vi "HFRR ADV v041.vi"() -> ()   [LabVIEW 2025] (continued)
  # "Step 2 — Disc Holder"
  # "Remove the disc holder by loosening and removing the opposing screws. Clean any fluid present in the disc holder."
  # "Step 3 — Calibration Head"
  # "Place the calibration holder in position and securely tighten the center screw."
  # "Step 4 — Calibration Holder"
  # "Place the calibration holder in position and tighten the two securing screws"
  # "Step 5 — Tare (Spring at Free Length)"
  # "Ensure the spring is at its contact (compressed) length — the micrometer head is in contact. Click Tare Sensor to zero the friction force baseline."
  # "Step 6 — Measure Friction Force"
  # "Run the Actual Test to measure Friction Force."
  # "Step 7 — CALIBRATION RESULT"
  # "Calibration completed successfully. The measured friction force is within the acceptable tolerance range of the factory calibration value."
  # "Calibration failed. The measured friction force differs from the factory calibration value . Please perform the calibration again."
  # "Spring Constant: k = 1.000 N/mm\nSpring force |F| = k Ч d"
  # "Calibrates the sample/bath temperature sensor. \nUsed for test specimen and lubricant temperature measurement."
  # "Calibrates the ambient air temperature sensor. \nUsed for environmental chamber monitoring."
  # "Set B\n60 °C\nHigh-point calibration"
  # "Set A\n0 °C\nIce-point calibration"
  # "Set B\n60 °C\nHigh-point calibration"
  # "Set A\n0 °C\nIce-point calibration"
  # "Select Temperature Sensor"
  # "Choose which temperature sensor you are calibrating. Both use the same two-\npoint procedure: 0 °C (ice-point) and 60 °C (high-point)."
  # "Step 1 — Reference Instrument Setup"
  # "Connect a calibrated reference to the DUT port. This calibration performs two sets: one at 0 °C and one at 60 °C."
  # "Set A\n0 °C\nIce-point calibration"
  # "Set B\n60 °C\nHigh-point calibration"
  # "Allow the temperature bath to stabilise for at least 2 minutes at each set-point before recording the reading."
  # "Step 2 — Set A:  0 °C Calibration"
  # "Connect the  0 °C reference connector. Wait for the temperature to stabilise. Once stable, and click Record Point."
  # "Step 3 — Set B:  60 °C Calibration"
  # "Connect the  60 °C reference connector. Wait for the temperature to stabilise. Once stable, and click Record Point."
  # "Sample Temperature Calibration Complete"
  # "Sample Temperature Calibration PASSED\nMax deviation 0.200 °C — within ±0.5 °C tolerance. Two-point correction applied (0 °C & 60 °C)."
  # "Sample  Temperature Calibration Failed\nmeasured Sample Temperature differs from the factory calibration value"
  # "Step 1 — Reference Instrument Setup"
  # "Connect a calibrated reference to the DUT port. This calibration performs two sets: one at 0 °C and one at 60 °C."
  # "Set A\n0 °C\nIce-point calibration"
  # "Set B\n60 °C\nHigh-point calibration"
  # "Allow the temperature bath to stabilise for at least 2 minutes at each set-point before recording the reading."
  # "Step 2 — Set A:  0 °C Calibration"
  # "Connect the  0 °C reference connector. Wait for the temperature to stabilise. Once stable, and click Record Point."
  # "Step 3 — Set B:  60 °C Calibration"
  # "Connect the  60 °C reference connector. Wait for the temperature to stabilise. Once stable, and click Record Point."
  # "Air Temperature Calibration Complete"
  # "Air Temperature Calibration PASSED\nMax deviation 0.200 °C — within ±0.5 °C tolerance. Two-point correction applied (0 °C & 60 °C)."
  # "Air  Temperature Calibration Failed\nmeasured Sample Temperature differs from the factory calibration value"
  # "System Control Commands\nS;1 - Starts the full automation cycle (Runs Priming-humidify till 70RH sequence first, then switches to Maintenance).\nS;0 - Stops the system immediately and enters Standby mode (Safe State: All actuators OFF).\nM;1 - Skips the priming sequence and jumps directly to Maintenance mode (PID control).\nR;1 - Resets the logic state machine and clears all errors, returning to Standby.\nService Mode (Manual Control)\nX;1 - Enters Manual Service Mode. This disables all automatic logic, sensor safety checks, and timers.\nX;0 - Exits Manual Service Mode and returns to Standby (Safe State).\nActuator Commands (Only work after sending X;1)\nP;[0-255] - Sets the Pump PWM. Note that this is Active Low (0 = Max Flow, 255 = Pump OFF).\nF;I;[0-255] - Sets the Intake Fan speed (0 = OFF, 255 = Max Speed).\nF;O;[0-255] - Sets the Exhaust Fan speed (0 = OFF, 255 = Max Speed).\nD;1 - Turns the Dehumidifier Relay ON.\nD;0 - Turns the Dehumidifier Relay OFF."
  # "%RH"
  # "ISO : WS1.4"
  # "Start test and end test log--- done\nDisable heater ON and Humidity ON during the test --- done\ntemprature and ---done\nhumidity reach log\nauto start run true logic and log\nmanual start log once"
  # "Reference Fluid Information"
  # "Note:\nMake sure to place all images in the folder \"C:\\WinDucom\\im\" before clicking on \"Import Image.\""
  # "NOTE:\nPlace all the images in the path \"C:\\WinDucom\\im\" before clicking on Import Image"
  # "Wear Scar Measurements"
  # "Reference Fluid Information"
  # "Graph :"
types:
  T1 = enum32{"Home", "Dashboard", "Imaging", "Report", "Analysis", "About", "Test Setup", "Advance", "Calibration"}
  T2 = enum32{"HOME", "Test Setup", "Acquire", "Adv Scar", "Adv Scar Report", "Compare Files", "Calibration", "About", "Advance", "Mooha"}
  T3 = enum16{"ASTM D6079", "ISO 12156", "CEC F-096-A-06", "Custom"}
  T4 = enum32{"Dashboard 1", "Dashboard 2", "Dashboard 3"}
  T5 = enum32{"COF", "Friction", "ECR", "Temperature", "Stroke"}
  T6 = enum32{"Coefficient Of Friction", "Air Temperature", "Humidity", "Stroke", "Sample Temperature", "Electrical Contact Resistance", "Frequency", "Air Temp vs Rh"}
  T7 = enum32{"Main", "Stroke", "Friction", "Temperature"}
  T8 = enum32{"Stroke Calibration", "Friction Force Calibration", "Temperature Calibration", "Default"}
  T9 = enum32{"Step 1", "Step 2", "Step 3", "Step 4", "Step 5", "Step 6", "Step 7", "Step 8", "Step 9"}
  T10 = enum32{"Test Progress", "Stroke Points Completed"}
  T11 = enum32{"Page 1", "Page 2", "Page 3", "Page 4", "Page 5", "Page 6", "Page 7"}
  T12 = enum32{"Main", "Step 1", "Step 2", "Step 3", "Step 4", "Air Step 1", "Air Step 2", "Air Step 3", "Air Step 4"}
  T13 = enum32{"Air Temperature", "Sample Temperature", "Default"}
  T14 = enum32{"COMMUNICATION", "CALIBRATION", "Temp Variables", "Camera", "WO 2465 (1)", "WO 2465 (2)", "WO 2465 (3)"}
  T15 = typedef "Auto Start enum.ctl" = enum16{"Init", "Humidity & Temperature On", "Reach point", "Maintain Stage", "Start Stage", "close", "Exit"}
  T16 = typedef "imagedata.ctl" = cluster{"image type":i32, "image depth":i32, "image":u8[], "mask":u8[], "colors":u32[], "Rectangle":cluster{"left":i16, "top":i16, "right":i16, "bottom":i16}}
  T17 = enum32{"HOME", "Test Setup", "Acquire", "Compare Files", "Print Report", "About", "Advance", "Mooha"}
  T18 = cluster{"Read Heave and Surge":string, "Bytes at Heave Port":dbl, "Heave and Surge COM Port:":refnum<visa-resource-name>, "Com Port 2":refnum<visa-resource-name>, "Residual Due":string, "Heave COM Status 2":bool, "Heave COM Status":bool, "Port 2":bool, "Sway PPR":dbl, "Surge PPR":dbl, "Heave PPR":dbl, "Sway Pitch":dbl, "Surge Pitch":dbl, "Heave Pitch":dbl, "Sway Pulses/mm":dbl, "Surge Pulses/mm":dbl, "Heave Pulses/mm":dbl, "inner loop":dbl, "Read Heave and Surge 2":string, "String 36":string, "Write S":bool, "WriteCC1":string[], "Heave COM Loop":i32, "LastCom":string, "EXIT":bool, "Error Heave":errorcluster}
  T19 = enum8{"Enabled", "Disabled", "Disabled and Grayed Out"}
  T20 = cluster{"Read Uno":string, "Bytes at Heave Port":dbl, "UNO COM Port:":refnum<visa-resource-name>, "UNO COM Port: 2":refnum<visa-resource-name>, "Residual Due":string, "UNO COM Status 2":bool, "UNO COM Status":bool, "Port 2":bool, "Sway PPR":dbl, "Surge PPR":dbl, "Heave PPR":dbl, "Sway Pitch":dbl, "Surge Pitch":dbl, "Heave Pitch":dbl, "Sway Pulses/mm":dbl, "Surge Pulses/mm":dbl, "Heave Pulses/mm":dbl, "inner loop":dbl, "Read Heave and Surge 2":string, "String 36":string, "Write S":bool, "WriteCC1":string[], "Heave COM Loop":i32, "LastCom":string, "EXIT":bool, "Error Heave":errorcluster}
  T21 = enum32{"HOME", "Test Setup", "Acquire", "Adv Scar", "Adv Scar Report", "Compare Files", "About", "Advance", "Mooha"}
  T22 = typedef "POST ANALYSIS ENUM.ctl" = enum16{"OPEN EXE", "INIT", "OPEN FILE", "FIT", "DRAW REC", "DRAW LINE", "PAN", "ZOOM IN", "ZOOM OUT", "SET ZOOM", "CLEAR ROI", "GET MEASUREMENTS", "RESIZE MODE", "STREAM START", "STREAM STOP", "SHOW UI", "MINIMIZE UI", "HIDE UI", "CKISE APP", "CLOSE CONNECTION", "SAVE IMAGE", "SET ROI COLOR", "READ", "TCP CHECK", "CLOSE"}
  T23 = typedef "CAMERA LIVE FEED ENUM.ctl" = enum16{"OPEN EXE", "INIT", "READ", "CAMERA CONNECT", "CAMERA START", "CAMERA STOP", "CAMERA GRAY", "CAMERA RGB", "CAMERA MINIMIZE", "CAMERA CLOSE", "CAMERA MODE LIST", "CAMERA MODE SET", "CAMERA RESTORE", "CAMERA SAVE", "CLOSE"}
  T24 = enum16{"Always On", "Always Off", "Off While Running"}
  T25 = enum32{"Page 1", "Page 2", "Page 3", "Page 4", "Page 5", "Page 6"}
  T26 = enum32{"Home", "Dashboard", "Imaging", "Report", "Analysis", "About", "Test Setup", "Advance"}
  T27 = cluster{"File Name":string, "Test Method":string, "Operator":string, "Fuel Description":string, "Date and time":string}
  T28 = enum32{"Home", "Dashboard", "Imaging", "Report", "Analysis", "About", "Test Setup"}
  T29 = enum32{"HOME", "Test Setup", "Acquire", "Compare Files", "About", "Advance", "Mooha"}
  T30 = typedef "NI_ReportGenerationCore.lvlib/HTML Report Image Alignment.ctl" = enum16{"(default)", "LEFT", "RIGHT", "TOP", "TEXTTOP", "MIDDLE", "ABSMIDDLE", "BASELINE", "BOTTOM", "ABSBOTTOM"}
  T31 = cluster{"y":dbl, "LVDT STROKE DISPLAY":dbl, "y":dbl}
  T32 = enum16{"INIT", "READ", "MANUAL WRITE", "WRITE", "CLOSE", "ERROR INIT"}
diagram:
  w5 = 0.0 ("ch0_filt")
  w7 = -9999999.0 ("max_ch0")
  w8 = 9999999.0 ("min_ch0")
  w19 = FALSE ("Visible")
  w20 = T19."Enabled" ("Disabled")
  w23 = FALSE ("Visible")
  w22 = FALSE ("Humidity Off Command")
  w38 = "" ("USER ID")
  (unwired) T21."HOME" ("Main Tab")
  # "Temperature Continue Air Step 2"
  # "[CH1]    - FF\n[CH2]   - TEMPERATURE\n[CH3]    - Humidity\n[CH4]    - AIR TEMP\n[CH5]\\- Visa Uno\n[CH6] \\- Visa Due\n[CH7]  \\- file path\n[CH8]   - Displacement Gain\n[CHA]   - Stroke Gain\n[CHB]   - Stroke PID Gain\n[CHC]   -Language Selection\n[CHD]   -Power +\n[CHE]   -Power_\n[CHF]   -Heater\n[CHG]   -Humidity Wet\n[CHH]   -Humidity Dry\n[CHI]   -Integral Time \n[CHIJ   -Air intercept\n[CHI]   -Temp Intercept"
  n1 = local write "Cal Password"("" ("Cal Password")) -> ()
  n2 = property on="Auto Start Test" class="Bool (strict)"("Visible"=TRUE) -> ()  [unwired: 2 in, 2 out]
  n3 = property on="FRICVALZ 2" class="Bool (strict)"("DisabledEnum"=w20) -> ()  [unwired: 2 in, 2 out]
  n4 = property on="FRICVALZ 4" class="Bool (strict)"("DisabledEnum"=w20) -> ()  [unwired: 2 in, 2 out]
  n5 = property on="FRICVALZ 3" class="Bool (strict)"("DisabledEnum"=w20) -> ()  [unwired: 2 in, 2 out]
  n6 = property on="About" class="Clust (strict)"("Visible"=FALSE) -> ()  [unwired: 2 in, 2 out]
  n7 = property on="Wrong Password" class="Str"("Visible"=w19) -> ()  [unwired: 2 in, 2 out]
  n8 = property on="Calibration 2" class="TabCtl (strict)"("Visible"=w19) -> ()  [unwired: 2 in, 2 out]
  n9 = local write "Temperature Selection"(T13."Default" ("Temperature Selection")) -> ()
  n10 = flat-sequence {
    tunnel: [w66] -> w4
    tunnel: [w111] -> w30
    tunnel: w4 -> [w106]
    tunnel: [w112] -> w32
    tunnel: w30 -> [w112]
    tunnel: w32 -> [w172]
    tunnel: [w172] -> w31
    tunnel: w31 -> [w203]
    tunnel: [w203] -> w41
    tunnel: w41 -> [w210]
    tunnel: [w216] -> w29
    tunnel: [w204] -> w28
    tunnel: [w258] -> w3
    tunnel: [w257] -> _
    tunnel: w29 -> [w257]
    tunnel: w28 -> [w258]
    frame #0 {
      n11 = call "CLOSE CONNECTION.vi"("error in (no error)"="error in (no error) 2") -> ("error out"=w71:errorcluster)  [unwired: 10 in]
      n12 = call <vilib>:"Clear Errors.vi"("error in (no error)"=w71) -> ("error out"=w70:errorcluster)  [unwired: 5 in, 1 out]
      n13 = disable-structure shown="Enabled" {
        disable-tunnel: w70 -> [w98 _]
        disable-tunnel: [w97 _] -> w69
        frame Enabled {
          n14 = call <userlib>:"Fit VI window to Largest Dec.vi"("error in (no error)"=w98, "border spacing (2 px)"=1) -> ("error out"=w101:errorcluster, "dup VI Ref"=w105:refnum<vi>)  [unwired: 4 in]
          n15 = invoke on="Invoke Node" class="VI" method="FP.Run-Time Position.Maximized"(reference=w105, error in=w101) -> (error out=w102:errorcluster)  [unwired: 2 in, 3 out]
          n16 = call <vilib>:"Clear Errors.vi"("error in (no error)"=w102) -> ("error out"=w104:errorcluster)  [unwired: 5 in, 1 out]
          n17 = control-ref of="This VI"() -> (w96:refnum<vi>)
          n18 = invoke on="Invoke Node" class="VI" method="Default Vals.Reinit All"(reference=w96, error in=w104) -> (reference out=w100:refnum<vi>, error out=w99:errorcluster)  [unwired: 1 in, 1 out]
          n19 = Close Reference(reference=w100, error in (no error)=w99) -> (error out=w97:errorcluster)
        }
        frame Disabled {
        }
      }
      n20 = call "Stall Data Flow.vim"("value in"=w69, "milliseconds to wait"=u32 2000) -> ("value out"=w68:errorcluster)  [unwired: 1 out]
      n21 = call "Read Config.vi"("error in (no error)"=w68) -> ("error out"=w66:errorcluster, "STROKE PARAMETERS"=w77:dbl[], "ADC PARAMETERS"=w78:dbl[], "PID  PARAMETERS"=w79:dbl[], "CALIBRATION PARAMETERS"=w64:string[], "Stroke Calibration"=w76:string)  [unwired: 5 in]
      n22 = Index Array(array=w77) -> (element #1=w94:dbl, element #2=w95:dbl)  [unwired: 2 in]
      n23 = Index Array(array=w64) -> (element #1=w63:string, element #2=w62:string, element #3=w61:string, element #4=w60:string, element #5=w59:string)  [unwired: 5 in]
      n24 = Index Array(array=w78) -> (element #1=w90:dbl, element #2=w91:dbl, element #3=w92:dbl, element #4=w93:dbl)  [unwired: 4 in]
      n25 = Index Array(array=w79) -> (element #1=w81:dbl, element #2=w82:dbl, element #3=w83:dbl, element #4=w84:dbl, element #5=w85:dbl, element #6=w86:dbl, element #7=w87:dbl, element #8=w88:dbl, element #9=w89:dbl)  [unwired: 9 in]
      n26 = local write "milliseconds to wait"(w81) -> ()
      n27 = local write "dt"(w82) -> ()
      n28 = local write "kp"(w83) -> ()
      n29 = local write "ki"(w84) -> ()
      n30 = local write "kd"(w85) -> ()
      n31 = local write "max_step_change"(w86) -> ()
      n32 = local write "max_amplitude"(w87) -> ()
      n33 = local write "min_amplitude"(w88) -> ()
      n34 = local write "startup_cmd"(w89) -> ()
      n35 = local write "VREF"(w90) -> ()
      n36 = local write "ADC_Resolution"(w91) -> ()
      n37 = local write "PIEZO_CAL_FACTOR"(w92) -> ()
      n38 = local write "NORMAL_FORCE"(w93) -> ()
      n39 = local write "STROKE FILTER"(w94) -> ()
      n40 = local write "Add up Stroke"(w95) -> ()
      n41 = local write "Machine Serial Number"(w59) -> ()
      n42 = local write "STROKE CALIBRATION"(w63) -> ()
      n43 = local write "FRICTION CALIBRATION"(w62) -> ()
      n44 = local write "TEMPERATURE CALIBRATION"(w61) -> ()
      n45 = Fract/Exp String To Number(string=w60) -> (number=w65:dbl)  [unwired: 3 in, 1 out]
      n46 = Spreadsheet String To Array(delimiter (Tab)=";", format string="", spreadsheet string=w76, array type (2D Dbl)=dbl[] []) -> (array=w80:dbl[])
      n47 = local write "Temperature diff"(w65) -> ()
      n48 = local write "calibration values"(w80) -> ()
    }
    frame #1 {
      n49 = property on="Auto Scar Check" class="Clust (strict)"("Visible"=TRUE) -> ()  [unwired: 2 in, 2 out]
      n50 = property on="Sign In" class="Bool (strict)"("DisabledEnum"=T19."Disabled" ("Disabled")) -> ()  [unwired: 2 in, 2 out]
      n51 = local write "sign in temp"(FALSE ("sign in temp")) -> ()
      n52 = call "dialog box.vi"("Status"="Before starting the test, verify that the microscope cable is connected.", "error in"=w106) -> ("error out"=w111:errorcluster)  [unwired: 8 in]
    }
    frame #2 {
      (unwired) TRUE ("Re-Initialise")
      # "kkkkk"
      # "C:\\Windows\\wndcm_pw_stdED hfrr.txt"
      # "C:\\LAB-IQ NXT"
      # "C:\\LAB-IQ NXT\\wndcm_pw_stdED hfrr.txt"
      # "password file"
      n53 = Current VI's Path() -> (path=w128:path)
      n54 = Strip Path(path=w128) -> (stripped path=w121:path)  [unwired: 1 out]
      n55 = local write "main tab sub"(enum32{"Page 1", "Page 2"}."Page 1" ("main tab sub")) -> ()
      n56 = local write "Main Tab Display"(T4."Dashboard 1" ("Main Tab Display")) -> ()
      n57 = local write "Main Tab"(T2."HOME" ("Main Tab")) -> ()
      n58 = Path To String(path=w121) -> (string=w123:string)
      n59 = Search/Split String(string=w123, search string/char (-)=".exe") -> (match + rest of string=w125:string)  [unwired: 1 in, 2 out]
      n60 = Match True/False String(2:".vi" ("false string"), 3:".exe" ("true string"), 4:w125) -> (0:w122:bool)  [unwired: 1 out]
      n61 = List Folder(path=path "C:/LAB-IQ" ("directory path"), pattern="*.txt") -> (filenames=w134:string[])  [unwired: 2 in, 3 out]
      n62 = case shown="True" w122 {
        tunnel: w121 -> [w143 w145]
        tunnel: [w143 w144] -> w119
        frame False {
        }
        frame True {
          n63 = Strip Path(path=w145) -> (stripped path=w144:path)  [unwired: 1 out]
        }
      }
      n64 = Search 1D Array(1D array=w134, element="wndcm_pw_stdED hfrr.txt") -> (index of element=w137:i32)  [unwired: 1 in]
      n65 = Equal?(x=w137, y=-1) -> (x = y?=w132:bool)
      n66 = Path To String(path=w119) -> (string=→"Gain path":string)
      n67 = case shown="True" w132 {
        frame False {
        }
        frame True {
          n68 = String To Byte Array(string="123\n") -> (unsigned byte array=w150:u8[])
          n69 = Array Size(array=w150) -> (size(s)=w149:i32)
          n70 = for {
            N: w149 -> [_]
            tunnel: w150 -> [w163]
            tunnel: [w160] -> w152 mode=indexing
            tunnel: w149 -> [w155]
            i -> [w153]
            n71 = Decrement(x=w155) -> (x-1=w156:i32)
            n72 = Index Array(array=w163, index=w153) -> (element=w162:u8)
            n73 = Equal?(x=w153, y=w156) -> (x = y?=w157:bool)
            n74 = Number To Decimal String(number=w162) -> (decimal integer string=w161:string)  [unwired: 1 in]
            n75 = Select(t="", s=w157, f="\r") -> (s? t:f=w154:string)
            n76 = Concatenate Strings(w161, w154) -> (w160:string)
          }
          n77 = local read "file path"() -> (w146:path)
          n78 = Concatenate Strings(w152) -> (w148:string)
          n79 = call <vilib>:"Write Characters To File.vi"("append to file? (new file:F)"=FALSE, "character string"=w148, "file path (dialog if empty)"=w146) -> ()  [unwired: 2 in, 1 out]
        }
      }
      n80 = local write "conststatus"(0.0 ("rpm value : 2")) -> ()
      n81 = local write "EVENT LOG"("") -> ()
      n82 = local write "COUNT"(0 ("COUNT")) -> ()
      n83 = local write "clk"(0.0 ("clk")) -> ()
      n84 = local write "Flag"(0.0 ("Flag")) -> ()
      n85 = local write "Lan flag"(0.0 ("Lan flag")) -> ()
      n86 = local write "Com flag"(u32 0 ("Com flag")) -> ()
      n87 = local write "refresh flag"(FALSE ("refresh flag")) -> ()
      "file path" <- path "C:/LAB-IQ/wndcm_pw_stdED hfrr.txt" ("file path")
      "FF buffer" <- dbl[] [] ("FF buffer")
    }
    frame #3 {
      # "C:\\WinDucom\\calibrate WO 2391.dcf"
      n88 = String To Path(string="C:\\LAB-IQ\\Image Calibrate v01.dcf") -> (path=w167:path)
      n89 = String To Path(string="C:\\LAB-IQ\\calibrate WO 2465.dcf") -> (path=w171:path)
      n90 = Open/Create/Replace File "Open File"(file path (use dialog)=w171) -> (refnum out=w170:refnum<file>)  [unwired: 5 in, 2 out]
      n91 = Open/Create/Replace File ("Open File")(file path (use dialog)=w167) -> (refnum out=w166:refnum<file>)  [unwired: 5 in, 2 out]
      n92 = for {
        N: 4 -> [_]
        tunnel: w166 -> [w178]
        i -> [w174]
        n93 = Read from Text File ("Read File")(file (use dialog)=w178) -> (text=w179:string)  [unwired: 3 in, 3 out]
        n94 = String Subset(string=w179, offset (0)=6, length (rest)=10 ("length (rest)")) -> (substring=w175:string)
        n95 = Fract/Exp String To Number(string=w175) -> (number=w173:dbl)  [unwired: 3 in, 1 out]
        n96 = case shown="3" w174 {
          tunnel: w173 -> [w180 w181 _ w182 _]
          frame 0 {
            n97 = local write "5x Gain"(w180) -> ()
          }
          frame 1 {
            n98 = local write "10x Gain"(w181) -> ()
          }
          frame 2 {
          }
          frame 3 {
            n99 = local write "100x gain"(w182) -> ()
          }
          frame 4, Default {
          }
        }
      }
      n100 = for {
        N: 24 -> [_]
        tunnel: w170 -> [w191]
        i -> [w185]
        (unwired) TRUE ("line mode (F)")
        n101 = Read from Text File "Read File"(file (use dialog)=w191) -> (text=w190:string)  [unwired: 3 in, 3 out]
        n102 = Match Pattern(string=w190, regular expression="]") -> (after substring=w188:string)  [unwired: 1 in, 3 out]
        n103 = String Subset(string=w190, offset (0)=5, length (rest)=10 ("length (rest)")) -> (substring=w183:string)
        n104 = Fract/Exp String To Number(string=w183) -> (number=w184:dbl)  [unwired: 3 in, 1 out]
        n105 = Match Pattern(string=w188, regular expression="-") -> (before substring=w186:string)  [unwired: 1 in, 3 out]
        n106 = case shown="18" w185 {
          tunnel: w184 -> [_ _ _ _ _ _ _ _ _ _ w198 _ _ _ _ _ _ _ _ _ _ _ _ _ _]
          tunnel: w186 -> [_ _ _ _ w194 w195 w196 _ _ _ _ _ _ _ _ _ _ _ _ _ w199 _ w200 w201 _]
          frame 0 {
          }
          frame 1 {
          }
          frame 2 {
          }
          frame 3 {
          }
          frame 4 {
            n107 = local write "Com Port 1"(w194) -> ()
          }
          frame 5 {
            n108 = local write "Com Port 2"(w195) -> ()
            n109 = local write "visa due"(w195) -> ()
          }
          frame 6 {
            n110 = String To Path(string=w196) -> (path=w197:path)
            n111 = local write "File Path"(w197) -> ()
          }
          frame 7 {
          }
          frame 8 {
          }
          frame 9 {
          }
          frame 10 {
            n112 = local write "Language Selection"(w198) -> ()
          }
          frame 11 {
          }
          frame 12 {
          }
          frame 13 {
          }
          frame 14 {
          }
          frame 15 {
          }
          frame 16 {
          }
          frame 17 {
          }
          frame 18 {
          }
          frame 21 {
          }
          frame 22 {
            n113 = local write "Com Port 3"(w199) -> ()
          }
          frame 23 {
          }
          frame 19 {
            n114 = local write "C3 :"(w200) -> ()
          }
          frame 20 {
            n115 = local write "Camera Port :"(w201) -> ()
          }
          frame 24, Default {
          }
        }
      }
    }
    frame #4 {
      n116 = Wait (ms)(milliseconds to wait=u32 1000) -> ()  [unwired: 1 out]
    }
    frame #5 {
      w219 = u32 2000 ("milliseconds to wait")
      w246 = u32 2000 ("milliseconds to wait")
      n117 = call "CAMERA LIVE FEED FGV.vi"("Enum - Menu"=CAMERA_LIVE_FEED_ENUM."OPEN EXE", "error in (no error)"=w210) -> ("error out"=w252:errorcluster)  [unwired: 8 in, 1 out]
      n118 = call "IMAGE ANALYSIS.vi"("Enum"=POST_ANALYSIS_ENUM."OPEN EXE", "error in"=w210) -> ("error out"=w207:errorcluster)  [unwired: 8 in, 1 out]
      n119 = call "Stall Data Flow.vim"("value in"=w252, "milliseconds to wait"=w246) -> ("value out"=w250:errorcluster)  [unwired: 1 out]
      n120 = call "Stall Data Flow.vim"("value in"=w207, "milliseconds to wait"=u32 8000) -> ("value out"=w206:errorcluster)  [unwired: 1 out]
      n121 = call "CAMERA LIVE FEED FGV.vi"("Enum - Menu"=CAMERA_LIVE_FEED_ENUM."INIT", "error in (no error)"=w250) -> ("error out"=w248:errorcluster)  [unwired: 8 in, 1 out]
      n122 = call "IMAGE ANALYSIS.vi"("Enum"=POST_ANALYSIS_ENUM."INIT", "error in"=w206) -> ("error out"=w204:errorcluster)  [unwired: 8 in, 1 out]
      n123 = case shown="Error .." w248 {
        selector: w248 -> [w253 _]
        tunnel: [w253 _] -> w247
        frame No Error {
        }
        frame Error {
          n124 = One Button Dialog(message="Camera initialization error.\nPlease Restart the software") -> ()  [unwired: 1 in, 1 out]
        }
      }
      n125 = property on="Camera Port :" class="CmbBox"() -> ("Strings[]"=w244:string[], "Value"=w245:string)  [unwired: 2 in, 2 out]
      n126 = Search 1D Array(1D array=w244, element=w245) -> (index of element=w243:i32)  [unwired: 1 in]
      n127 = Type Cast(type=30, x=w243) -> (*(type *) &x=w241:i32)
      n128 = call "Stall Data Flow.vim"("value in"=w247, "milliseconds to wait"=w246) -> ("value out"=w223:errorcluster)  [unwired: 1 out]
      n129 = Add(x=w241, y=48) -> (x+y=w222:i32)
      n130 = call "CAMERA LIVE FEED FGV.vi"("Enum - Menu"=CAMERA_LIVE_FEED_ENUM."CAMERA CONNECT", "error in (no error)"=w223, "CAMERA PORT"=w222) -> ("error out"=w232:errorcluster)  [unwired: 7 in, 1 out]
      n131 = call "Stall Data Flow.vim"("value in"=w232, "milliseconds to wait"=u32 5000) -> ("value out"=w233:errorcluster)  [unwired: 1 out]
      n132 = call "CAMERA LIVE FEED FGV.vi"("Enum - Menu"=CAMERA_LIVE_FEED_ENUM."CAMERA MODE LIST", "error in (no error)"=w233) -> ("error out"=w235:errorcluster)  [unwired: 8 in, 1 out]
      n133 = call "Stall Data Flow.vim"("value in"=w235, "milliseconds to wait"=w219) -> ("value out"=w234:errorcluster)  [unwired: 1 out]
      n134 = call "CAMERA LIVE FEED FGV.vi"("Enum - Menu"=CAMERA_LIVE_FEED_ENUM."READ", "error in (no error)"=w234) -> ("error out"=w221:errorcluster, "data out"=→"Camera List":string)  [unwired: 8 in]
      n135 = Type Cast(type=30, x=0) -> (*(type *) &x=w215:i32)
      n136 = call "Stall Data Flow.vim"("value in"=w221, "milliseconds to wait"=w219) -> ("value out"=w220:errorcluster)  [unwired: 1 out]
      n137 = Add(x=w215, y=48) -> (x+y=w213:i32)
      n138 = call "CAMERA LIVE FEED FGV.vi"("Enum - Menu"=CAMERA_LIVE_FEED_ENUM."CAMERA MODE SET", "error in (no error)"=w220, "CAMERA MODE"=w213) -> ("error out"=w217:errorcluster)  [unwired: 7 in, 1 out]
      n139 = call "Stall Data Flow.vim"("value in"=w217, "milliseconds to wait"=u32 2000) -> ("value out"=w237:errorcluster)  [unwired: 1 out]
      n140 = call "CAMERA LIVE FEED FGV.vi"("Enum - Menu"=CAMERA_LIVE_FEED_ENUM."CAMERA START", "error in (no error)"=w237) -> ("error out"=w238:errorcluster)  [unwired: 8 in, 1 out]
      n141 = call "Stall Data Flow.vim"("value in"=w238, "milliseconds to wait"=u32 1000) -> ("value out"=w239:errorcluster)  [unwired: 1 out]
      n142 = call "CAMERA LIVE FEED FGV.vi"("Enum - Menu"=CAMERA_LIVE_FEED_ENUM."CAMERA MINIMIZE", "error in (no error)"=w239) -> ("error out"=w216:errorcluster)  [unwired: 8 in, 1 out]
    }
    frame #6 {
      n143 = case shown="No Error" w257 {
        frame No Error {
          n144 = property on="Auto Scar Check" class="Clust (strict)"("Visible"=FALSE) -> ()  [unwired: 2 in, 2 out]
        }
        frame Error {
        }
      }
      n145 = property on="Sign In" class="Bool (strict)"("DisabledEnum"=T19."Enabled" ("Disabled")) -> ()  [unwired: 2 in, 2 out]
      n146 = local write "sign in temp"(TRUE ("sign in temp")) -> ()
    }
  }
  n147 = local write "Calibration Selection"(T8."Default" ("Calibration Selection")) -> ()
  n148 = local write "SCAR MEASURMENT"(enum32{"Auto Scar", "Manual Scar"}."Manual Scar" ("SCAR MEASURMENT")) -> ()
  n149 = local write "Temperature Off Command"(w22) -> ()
  n150 = local write "Main Dashboard Buttons"(T1."Home" ("Main Dashboard Buttons")) -> ()
  n151 = local write "Humidity Off Command"(w22) -> ()
  n152 = local write "CAMERA ROI MIN TEMP"(w22) -> ()
  n153 = local write "TEST FILE NAM,E SAVED"(w22) -> ()
  n154 = local write "LIVE FEED MIN TEMP"(w22) -> ()
  n155 = local write "SCAR MEASURMENT"(enum32{"Auto Scar", "Manual Scar"}."Manual Scar" ("SCAR MEASURMENT")) -> ()
  n156 = local write "Auto stop temp"(w23) -> ()
  n157 = local write "main tab sub"(enum32{"Page 1", "Page 2"}."Page 1" ("main tab sub")) -> ()
  n158 = while {
    stop <- w272 stop-if-true
    n159 = local read "Ambient Temperature"() -> (w270:dbl)
    n160 = local read "Sample Temperature"() -> (w269:dbl)
    n161 = Wait (ms)(milliseconds to wait=u32 200) -> ()  [unwired: 1 out]
    n162 = local write "Sensor value"(w270) -> ()
    n163 = local write "Sensor value"(w270) -> ()
    n164 = local write "Sensor value"(w269) -> ()
    n165 = local write "Sensor value"(w269) -> ()
    n166 = local write "Temperature — Live (Set A: 0 °C)"(w270) -> ()
    n167 = local write "Temperature — Live (Set A: 60 °C)"(w270) -> ()
    n168 = local write "Temperature — Live (Set A: 60 °C)"(w269) -> ()
    n169 = local write "Temperature — Live (Set A: 0 °C)"(w269) -> ()
    n170 = case shown="True" "Save Button" {
      selector: "Save Button" -> [_ w322]
      frame False {
      }
      frame True {
        n171 = local read "Temperature diff"() -> (w318:dbl)
        n172 = local read "Machine Serial Number"() -> (w307:string)
        n173 = Not(x=w322) -> (.not. x?=w321:bool)
        n174 = local read "milliseconds to wait"() -> (w354:u32)
        n175 = local read "max_step_change"() -> (w359:dbl)
        n176 = local read "max_amplitude"() -> (w360:dbl)
        n177 = local read "min_amplitude"() -> (w361:dbl)
        n178 = local read "PIEZO_CAL_FACTOR"() -> (w365:dbl)
        n179 = local write "Save Button"(w321) -> ()
        n180 = local read "startup_cmd"() -> (w362:dbl)
        n181 = local read "NORMAL_FORCE"() -> (w366:dbl)
        n182 = local read "ADC_Resolution"() -> (w364:dbl)
        n183 = local read "calibration values"() -> (w369:dbl[])
        n184 = local read "kp"() -> (w356:dbl)
        n185 = local read "kd"() -> (w358:dbl)
        n186 = local read "dt"() -> (w355:dbl)
        n187 = local read "ki"() -> (w357:dbl)
        n188 = local read "STROKE FILTER"() -> (w367:i32)
        n189 = local read "Add up Stroke"() -> (w368:dbl)
        n190 = Number To Fractional String(number=w318) -> (F-format string=w317:string)  [unwired: 3 in]
        n191 = local read "VREF"() -> (w363:dbl)
        n192 = Insert Into Array(array=dbl[] [], new element #1=w354, new element #2=w355, new element #3=w356, new element #4=w357, new element #5=w358, new element #6=w359, new element #7=w360, new element #8=w361, new element #9=w362) -> (w370:dbl[])  [unwired: 1 in]
        n193 = Insert Into Array(array=dbl[] [], new element #1=w363, new element #2=w364, new element #3=w365, new element #4=w366) -> (w371:dbl[])  [unwired: 1 in]
        n194 = Array To Spreadsheet String(delimiter (Tab)=";", array=w369, 3:"" ("format string")) -> (spreadsheet string=w373:string)
        n195 = Insert Into Array(array=dbl[] [], new element #1=w367, new element #2=w368) -> (w372:dbl[])  [unwired: 1 in]
        n196 = Insert Into Array(array=string[] [], new element #1="STROKE CALIBRATION", new element #2="FRICTION CALIBRATION", new element #3="TEMPERATURE CALIBRATION", new element #4=w317, new element #5=w307) -> (w319:string[])  [unwired: 1 in]
        n197 = call "Write Config.vi"("Stroke Calibration"=w373, "CALIBRATION PARAMETERS"=w319, "STROKE PARAMETERS"=w372, "ADC PARAMETERS"=w371, "PID  PARAMETERS"=w370) -> ("error out"=w352:errorcluster)  [unwired: 6 in]
        n198 = call "Stall Data Flow.vim"("value in"=w352, "milliseconds to wait"=u32 2000) -> ("value out"=w353:errorcluster)  [unwired: 1 out]
        n199 = call "Read Config.vi"("error in (no error)"=w353) -> ("STROKE PARAMETERS"=w350:dbl[], "ADC PARAMETERS"=w349:dbl[], "PID  PARAMETERS"=w348:dbl[], "CALIBRATION PARAMETERS"=w313:string[], "Stroke Calibration"=w351:string)  [unwired: 5 in, 1 out]
        n200 = Index Array(array=w348) -> (element #1=w346:dbl, element #2=w345:dbl, element #3=w344:dbl, element #4=w343:dbl, element #5=w342:dbl, element #6=w341:dbl, element #7=w340:dbl, element #8=w339:dbl, element #9=w338:dbl)  [unwired: 9 in]
        n201 = Index Array(array=w349) -> (element #1=w337:dbl, element #2=w336:dbl, element #3=w335:dbl, element #4=w334:dbl)  [unwired: 4 in]
        n202 = Index Array(array=w350) -> (element #1=w333:dbl, element #2=w332:dbl)  [unwired: 2 in]
        n203 = Index Array(array=w313) -> (element #1=w310:string, element #2=w309:string, element #3=w308:string, element #4=w312:string, element #5=w306:string)  [unwired: 5 in]
        n204 = Spreadsheet String To Array(delimiter (Tab)=";", format string="", spreadsheet string=w351, array type (2D Dbl)=dbl[] []) -> (array=w347:dbl[])
        n205 = local write "VREF"(w337) -> ()
        n206 = local write "ADC_Resolution"(w336) -> ()
        n207 = local write "PIEZO_CAL_FACTOR"(w335) -> ()
        n208 = local write "NORMAL_FORCE"(w334) -> ()
        n209 = local write "STROKE CALIBRATION"(w310) -> ()
        n210 = local write "FRICTION CALIBRATION"(w309) -> ()
        n211 = local write "TEMPERATURE CALIBRATION"(w308) -> ()
        n212 = Fract/Exp String To Number(string=w312) -> (number=w311:dbl)  [unwired: 3 in, 1 out]
        n213 = local write "Machine Serial Number"(w306) -> ()
        n214 = local write "STROKE FILTER"(w333) -> ()
        n215 = local write "Add up Stroke"(w332) -> ()
        n216 = local write "calibration values"(w347) -> ()
        n217 = local write "milliseconds to wait"(w346) -> ()
        n218 = local write "dt"(w345) -> ()
        n219 = local write "kp"(w344) -> ()
        n220 = local write "ki"(w343) -> ()
        n221 = local write "kd"(w342) -> ()
        n222 = local write "max_step_change"(w341) -> ()
        n223 = local write "max_amplitude"(w340) -> ()
        n224 = local write "min_amplitude"(w339) -> ()
        n225 = local write "startup_cmd"(w338) -> ()
        n226 = local write "Temperature diff"(w311) -> ()
      }
    }
    n227 = local read "USER ID"() -> (w267:string)
    n228 = local read "run test Calibration"() -> (w265:bool)
    n229 = disable-structure shown="Enabled" {
      disable-tunnel: [w277 w288] -> w266
      frame Disabled {
        n230 = local read "Point 1 - 0.2 mm"() -> (w287:bool)
        n231 = local read "Point 2 - 0.4 mm"() -> (w286:bool)
        n232 = local read "Point 3 - 0.6 mm"() -> (w285:bool)
        n233 = local read "Point 4 - 0.8 mm"() -> (w284:bool)
        n234 = local read "Point 5 - 1.0 mm"() -> (w283:bool)
        n235 = local read "Point 6 - 1.2 mm"() -> (w282:bool)
        n236 = And(x=w287, y=w286) -> (x .and. y?=w281:bool)
        n237 = And(x=w285, y=w284) -> (x .and. y?=w280:bool)
        n238 = And(x=w283, y=w282) -> (x .and. y?=w278:bool)
        n239 = And(x=w281, y=w280) -> (x .and. y?=w279:bool)
        n240 = And(x=w279, y=w278) -> (x .and. y?=w277:bool)
      }
      frame Enabled {
        n241 = local read "Point 5 - 1.0 mm"() -> (w288:bool)
      }
    }
    n242 = local read "START TEMP"() -> (w264:bool)
    n243 = local write "tested by 2"(w267) -> ()
    n244 = And(x=w264, y=w265) -> (x .and. y?=w263:bool)
    n245 = case shown="True" w263 {
      frame False {
        w289 = TRUE ("PAUSE")
        n246 = call "ELAPSED TIMER VI - Calibration.vi"("RESET"=w289, "PAUSE"=w289) -> ()  [unwired: 7 in, 3 out]
      }
      frame True {
        w292 = FALSE ("PAUSE")
        n247 = call "ELAPSED TIMER VI - Calibration.vi"("TARGET"=60.0, "RESET"=w292, "PAUSE"=w292) -> ("ELAPSED INDICATION"=w290:bool)  [unwired: 6 in, 2 out]
        n248 = case shown="True" w290 {
          frame False {
            n249 = local write "Friction Force Calibration Result Tab"(enum32{"Calibration Results", "Page 2"}."Calibration Results" ("Friction Force Calibration Result Tab")) -> ()
            n250 = property on="Friction Force Calibration Result Tab" class="TabCtl (strict)"("Visible"=TRUE) -> ()  [unwired: 2 in, 2 out]
          }
          frame True {
            n251 = stacked-sequence {
              frame #0 {
                n252 = local read "Friction"() -> (→"Friction cal":dbl)
                n253 = local write "START TEMP"(FALSE ("START TEMP")) -> ()
              }
              frame #1 {
                n254 = Wait (ms)(milliseconds to wait=u32 1500) -> ()  [unwired: 1 out]
              }
              frame #2 {
                n255 = local write "Due Write"("VC;0") -> ()
              }
              frame #3 {
                n256 = Wait (ms)(milliseconds to wait=u32 1500) -> ()  [unwired: 1 out]
              }
              frame #4 {
                n257 = local write "Due Write"("VC;0") -> ()
              }
              frame #5 {
                n258 = property on="Friction Force Calibration Result Tab" class="TabCtl (strict)"("Visible"=TRUE) -> ()  [unwired: 2 in, 2 out]
              }
            }
          }
        }
      }
    }
    n259 = local read "Friction cal"() -> (w262:dbl)
    n260 = case shown="False" w266 {
      frame False {
        n261 = property on="Accept & Save" class="Bool (strict)"("DisabledEnum"=T19."Disabled" ("Disabled")) -> ()  [unwired: 2 in, 2 out]
        n262 = property on="Tab Control 5" class="TabCtl (strict)"("Value"=enum32{"OK", "NG"}."NG" ("Tab Control 5")) -> ()  [unwired: 2 in, 2 out]
      }
      frame True {
        n263 = property on="Accept & Save" class="Bool (strict)"("DisabledEnum"=T19."Enabled" ("Disabled")) -> ()  [unwired: 2 in, 2 out]
        n264 = property on="Tab Control 5" class="TabCtl (strict)"("Value"=enum32{"OK", "NG"}."OK" ("Tab Control 5")) -> ()  [unwired: 2 in, 2 out]
      }
    }
    n265 = Greater Or Equal?(x=w262, y="FF CAL EXCPTED VALUE") -> (x >= y?=w260:bool)
    n266 = case shown="True" w260 {
      frame False {
        n267 = local write "Friction Force result Tab"(enum32{"OK", "NG"}."NG" ("Friction Force result Tab")) -> ()
        n268 = property on="Accept & Save FF" class="Bool (strict)"("DisabledEnum"=T19."Disabled" ("Disabled")) -> ()  [unwired: 2 in, 2 out]
      }
      frame True {
        n269 = local write "Friction Force result Tab"(enum32{"OK", "NG"}."OK" ("Friction Force result Tab")) -> ()
        n270 = property on="Accept & Save FF" class="Bool (strict)"("DisabledEnum"=T19."Enabled" ("Disabled")) -> ()  [unwired: 2 in, 2 out]
      }
    }
    n271 = local read "Quit"() -> (w272:bool)
  }
  n272 = local write "USERNAME"(w38) -> ()
  n273 = local write "Main Tab"(T2."HOME" ("Main Tab")) -> ()
  n274 = local write "USER ID"(w38) -> ()
  n275 = property on="Auto Scar Check  2" class="Clust (strict)"("Visible"=w23) -> (error out=w26:errorcluster)  [unwired: 2 in, 1 out]
  n276 = property on="Quit" class="Bool (strict)"("Value"=FALSE ("Quit")) -> (error out=w40:errorcluster)  [unwired: 2 in, 1 out]
  n277 = while {
    stop <- w374 stop-if-true
    n278 = event shown="[2] \"run test Calibration\": Value Change" {
      selector: _ -> [_ _ _ _ _ _ _ _ _ _ _ _ _ _ _ _ _ _ _ _ _ _ _ _ _ _ _ _ _ _ _ _ _ _ _ _ _ _ _ _ _ _ _ _ _ _ _ _ _ _ _ _ _ _ _]
      dyn-events: _ -> [_ _ _ _ _ _ _ _ _ _ _ _ _ _ _ _ _ _ _ _ _ _ _ _ _ _ _ _ _ _ _ _ _ _ _ _ _ _ _ _ _ _ _ _ _ _ _ _ _ _ _ _ _ _ _]
      timeout: 100 -> [_ _ _ _ _ _ _ _ _ _ _ _ _ _ _ _ _ _ _ _ _ _ _ _ _ _ _ _ _ _ _ _ _ _ _ _ _ _ _ _ _ _ _ _ _ _ _ _ _ _ _ _ _ _ _]
      tunnel: [FALSE FALSE FALSE _ FALSE _ _ _ _ _ _ _ _ _ _ _ _ _ _ _ _ _ _ _ _ _ _ _ _ _ _ _ _ _ _ _ _ _ _ _ _ _ _ _ _ _ _ _ _ _ _ _ _ _ TRUE] -> w374
      event Timeout {
        n279 = event-data() -> ()  [unwired: 1 in, 3 out]
        n280 = disable-structure shown="Disabled" {
          frame Disabled {
            n281 = local read "Auto Start Test"() -> (w388:bool)
            n282 = local read "RUN"() -> (w389:bool)
            n283 = Or(x=w389, y=w388) -> (x .or. y?=w387:bool)
            n284 = case shown="True" w387 {
              frame False {
                w390 = TRUE ("PAUSE")
                n285 = call "ELAPSED TIMER VI - abort test.vi"("RESET"=w390, "PAUSE"=w390) -> ()  [unwired: 7 in, 3 out]
              }
              frame True {
                n286 = local read "Stroke 2"() -> (w395:dbl)
                n287 = local read "FF 3"() -> (w397:dbl)
                n288 = Equal?(x=w395, y=0.95 ("Stroke 2")) -> (x = y?=w392:bool)
                n289 = Equal?(x=w397, y=0.0 ("FF 3")) -> (x = y?=w393:bool)
                n290 = Or(x=w393, y=w392) -> (x .or. y?=w391:bool)
                n291 = case shown="True" w391 {
                  selector: w391 -> [_ w402]
                  frame False {
                    w398 = TRUE ("PAUSE")
                    n292 = call "ELAPSED TIMER VI - abort test.vi"("RESET"=w398, "PAUSE"=w398) -> ()  [unwired: 7 in, 3 out]
                  }
                  frame True {
                    n293 = Not(x=w402) -> (.not. x?=w401:bool)